vi "UHR-Fleezers Control (host) - Avogadro v2.vi"() -> ()   [LabVIEW 2014] (continued)
  in  "Clear Volume P3":bool caption="Clear Infused Volume"
  in  "Clear Volume P1":bool caption="Clear Infused Volume"
  in  "Display On P1":bool caption="Display On"
  in  "All Pump Parameters":T14={"Pump 1"={"Diameter (mm)"=4.61, "Units"=4.0, "Volume"=100.0, "Rate"=25.0}, "Pump 2"={"Diameter (mm)"=4.61, "Units"=3.0, "Volume"=0.0, "Rate"=0.0}, "Pump 3"={"Diameter (mm)"=4.61, "Units"=4.0, "Volume"=100.0, "Rate"=800.0}}
  in  "Total Volume\nFlushed (uL)":dbl
  in  "Inject Pump 2":bool caption="Inject Pump 2\n(Flush Center)"
  in  "Flush Center Ch Rate (ul/m)":dbl=100.0
  in  "Flush Center Ch Volume (uL)":dbl=15.0
  in  "Pump pause delay (ms)":u32
  in  "Pump write delay (ms)":dbl=300.0
  in  "Ch 3 Inject Rate (ul/h)":dbl=800.0
  in  "Ch 3 Inject Volume (uL)":dbl=100.0
  in  "Ch 1 Inject Volume (uL)":dbl=100.0
  in  "Ch 1 Inject Rate (ul/h)":dbl=25.0
  out "Pump 1 cont disp":string="Right: DNA beads "
  out "Pump 3 cont disp":string="Left: ADig beads"
  in  "Read Harvard":bool
  out "read buffer":string
  out "Serial Settings:Number of Bytes at Serial Port":u32
  in  "write buffer":string
  in  "Tab Control 2":T15(tab)=enum."Feedback on Trap Intensity"
  in  "RF BD 2 to green AOM":bool=TRUE
  in  "RF synth green feedback max":i16=1300
  in  "Phase Increment Trap 2":fxp<+,14,14>=165.0
  in  "Phase offset method":u8=3
  in  "Phase Increment Trap 1":fxp<+,14,14>=165.0
  in  "RF phase reset before cycles":bool
  in  "Update all trap values":bool
  out "Total Counts (ticks)":u16=400
  in  "Trap ON/OFF X or Y Amp?":bool=TRUE
  in  "Oscillate Set 1":bool
  in  "Trap 1 ON":bool=TRUE
  in  "Number Interlace Sets":u8=2 min=1 max=3
  in  "DIO count 3 (ticks)":u16=200
  in  "DIO count 2 (ticks)":u16=200
  in  "DIO count 1 (ticks)":u16=200
  in  "BD 2 Amplitude 3 (%)":dbl min=0.0 max=45.0 step=1.0
  in  "BD 2 Amplitude 2 (%)":dbl min=0.0 max=45.0 step=1.0
  in  "BD 2 Amplitude 1 (%)":dbl min=0.0 max=45.0 step=1.0
  in  "BD 1 Amplitude 3 (%)":dbl min=0.0 max=50.0 step=1.0
  in  "BD 1 Amplitude 2 (%)":dbl=44.0 min=0.0 max=50.0 step=1.0
  in  "BD 1 Amplitude 1 (%)":dbl=45.0 min=0.0 max=50.0 step=1.0
  in  "BD 2 Frequency 3 (MHz)":dbl=26.0 min=0.0 max=40.0 step=0.1 format="%#_6p"
  in  "BD 1 Frequency 3 (MHz)":dbl=70.0 min=60.0 max=90.0 step=1.0 format="%#_6p"
  in  "BD 2 Frequency 2 (MHz)":dbl=26.0 min=0.0 max=40.0 step=0.1 format="%#_6p"
  in  "BD 2 Frequency 1 (MHz)":dbl=26.0 min=0.0 max=40.0 step=0.1 format="%#_6p"
  in  "Not-Interlacing Set":enum32{"Set 1", "Set 2", "Set 3"}(radio)
  in  "Interlace":bool=TRUE
  in  "Trap 2 ON":bool=TRUE
  in  "Trap 3 ON":bool
  in  "Scan axis 2":bool=TRUE
  in  "Osc. amp. (MHz)":dbl=2.0
  in  "Next trap write delay (ticks)":u8
  in  "Manipulation Scaling":cluster{"Horizontal":dbl, "Vertical":dbl}={"Horizontal"=0.075, "Vertical"=0.01}
  out "Coords":T16
  in  "RF amplitude switch delay":u16=2
  in  "BD 1 Delay (ticks)":u8=9
  in  "BD 2 Delay (Ticks)":u8
  in  "Swap F1 and F2":bool
  in  "MCL Step Increment (V_int)":dbl=3.0
  out "Time to Finish All (min)":dbl=0.20000000000000004 format="%#_2p"
  in  "Scan Speed (nm/s)":dbl=50.0
  in  "Scan Range (nm)":dbl=300.0
  in  "Step Size (nm)":dbl=1.0
  in  "MCL/AOM Scale Tweak":dbl=1.0
  in  "MCL Step Position Ratio":dbl=0.5
  in  "Move MCL Also?":bool
  out "Final sep (nm)":dbl=1641.7733990147785
  out "Initial sep (nm)":dbl=1460.0
  out "Save index":dbl=17.0
  out "Final delta (MHz)":dbl=21.477832512315274
  out "Initial delta (MHz)":dbl=20.0
  out "Final freq. (MHz)":dbl=68.52216748768473
  out "Initial freq. (MHz)":dbl=70.0
  in  "Saved AOD Raster Scan Parameter Sets":T17(array[cluster])=[{"Scan Range AOD (nm) 2"=2000.0, "Step Size AOD (nm) 2"=1.0, "Scan Speed AOD (nm/s) 2"=500.0, "Number of scans (AOD) 2"=1, "Label"="offset curve"}, {"Scan Range AOD (nm) 2"=450.0, "Step Size AOD (nm) 2"=1.0, "Scan Speed AOD (nm/s) 2"=100.0, "Number of scans (AOD) 2"=1, "Label"="hp raster check"}, {"Scan Range AOD (nm) 2"=6.8, "Step Size AOD (nm) 2"=0.34, "Scan Speed AOD (nm/s) 2"=0.34, "Number of scans (AOD) 2"=1, "Label"="3.4 kbp - 1 bp steps"}, {"Scan Range AOD (nm) 2"=200.0, "Step Size AOD (nm) 2"=1.0, "Scan Speed AOD (nm/s) 2"=50.0, "Number of scans (AOD) 2"=1, "Label"="dt14 1 14 MHz start"}, {"Scan Range AOD (nm) 2"=450.0, "Step Size AOD (nm) 2"=1.0, "Scan Speed AOD (nm/s) 2"=100.0, "Number of scans (AOD) 2"=1, "Label"="dt14 2 small beads"}, {"Scan Range AOD (nm) 2"=300.0, "Step Size AOD (nm) 2"=1.0, "Scan Speed AOD (nm/s) 2"=100.0, "Number of scans (AOD) 2"=1, "Label"="Oligo"}]
  in  "Load parameters":bool
  out "Scan Range (MHz)":dbl=-1.477832512315271
  in  "Restart DMA? (AOD)":bool=TRUE caption="Restart DMA?"
  out "Incr. int (AOD)":i64=-4701660970
  out "Time/Scan (s) (AOD)":dbl=6.000000000000001 format="%#_2p"
  out "Data points/scans":dbl=1200000.0
  out "Data points/scan (f/b)":dbl=1200000.0
  in  "Save scans":bool=TRUE
  out "AOD Scan I":u64=1 caption="Scan I"
  in  "Continuous AOD Scanning":bool caption="Continuous Scanning"
  in  "Abort AOD Scan":bool caption="Abort Scan"
  in  "Scan BD":bool=TRUE
  out "Cycles/step (AOD)":u64=2000 format="%.3p"
  in  "Number of F/B Scans (AOD)":u16=1 min=1
  out "Scan steps (AOD)":u64=300
  out "Scan Increment (MHz)":dbl=-0.004942583653228331
  out "AOD Scanning":bool caption="Scanning"
  in  "Start AOD Scan":bool caption="Start Scan"
  out "N sets should be saved":dbl=60.0
  out "Progress 2":u16(slide) caption="Progress" scale=0.0..100.0
  in  "Abort save 2":bool caption="Abort save"
  out "MCL Count":dbl=60182.50068666645
  out "T2 feedback amplitude":dbl
  out "T1 feedback amplitude":dbl
  in  "Trap intensity output range":cluster{"Normal High":i16, "Normal Low":i16}={"Normal High"=3000, "Normal Low"=0}
  in  "All FB On/Off":bool
  in  "AI2 to Setpoint":cluster{"Set 1":bool, "Set 2":bool}
  out "AI2 (V)":cluster{"Set 1":dbl, "Set 2":dbl}={"Set 1"=1.9983520004882962, "Set 2"=1.9980468153935362}
  in  "Reset Feedback":cluster{"Set 1":bool, "Set 2":bool}
  in  "Trap Intensity PID Gains":T18={"proportional gain (Kc)"=10, "integral gain (Kc*Ts/Ti)"=5, "derivative gain (Kc*Td/Ts)"=0}
  in  "Feedback On/Off":cluster{"Set 1":bool, "Set 2":bool}={"Set 1"=TRUE, "Set 2"=TRUE}
  out "Actual Setpoint":fxp<+/-,16,1> format="%.16g"
  in  "Dynamic Force FB (ronen)":bool=TRUE
  in  "Remove Unwinding Offset":bool
  in  "Set Reading to\nSetpoint":bool
  out "Trap X (AI1)":T19={"Trap 1"=-0.00103759765625, "Trap 2"=0.0006103515625}
  in  "Trap Pos FB SP":fxp<+/-,16,1>=0.009033203125 caption="Setpoint"
  in  "Trap Pos. FB ON":bool
  in  "Reset Trap Pos. FB":bool
  in  "Tab Control 8":T20(tab)=enum."Dynamic FB settings"
  in  "Red Laser ON/OFF":bool
  in  "Green Laser ON/OFF":bool
  in  "Offset SP2 from SP1":bool
  in  "Use SP 2":bool
  in  "Trap Pos FB Int Count":u16=100
  in  "Trap Pos. FB Gains":T21={"proportional gain (Kc)"=20.0, "integral gain (Kc*Ts/Ti)"=3.0, "derivative gain (Kc*Td/Ts)"=0.0} {"proportional gain (Kc)" format="%.11g"; "integral gain (Kc*Ts/Ti)" format="%.11g"; "derivative gain (Kc*Td/Ts)" format="%.11g"}
  in  "Trap Pos FB SP 2":fxp<+/-,16,1>=-0.10723876953125 caption="Setpoint 2"
  in  "SP2 Offset":fxp<+/-,16,1>=0.100006103515625
  in  "Blue Laser ON/OFF":bool
  in  "Negate Diff?":bool=TRUE
  in  "Differential FB?":bool=TRUE
  in  "Trap Pos. FB Offset Factor":i64
  in  "Trap Pos FB Negate Action":bool=TRUE
  in  "Trap Pos. FB Mult Factor":i64=8388608
  in  "Trap Pos. AI1 X Pre-scale":u16
  in  "Trap Pos. FB Range":T22={"output high"=0.999969482421875, "output low"=-1.0}
  out "Trap Pos FB Int Signal":fxp<+/-,24,9>=0.107635498046875 format="%.18g"
  out "Trap Pos FB Int-Norm Signal":fxp<+/-,16,1>=0.001068115234375 format="%.16g"
  in  "Set SP Using...":bool
  in  "Trap Pos FB Monitor\nT1 or T2":bool
  out "Trap X AI1 (DMA)":T23={"Set 1"=0.001190185546875, "Set 2"=-0.000396728515625}
  in  "N El. to Ave.":dbl=10000.0
  out "Trap Pos FB Action":i64
  in  "Target Force (pN)":dbl
  in  "Read Setpoint Correction File":bool
  out "Offset corrected setpoint":fxp<+/-,17,2>
  in  "Real time Offset file correction for setpoint":bool
  out "B factor":dbl=1.024047487221734
  out "Setpoint offset\ncorrection values":dbl[](array[numeric])=[-0.031124917445190622, -0.030752651903868396, -0.030380386362546155, -0.030008120821223914, -0.0296358552799017, -0.029263589738579454, -0.028891324197257227, -0.02851905865593498, -0.028146793114612746, -0.027774527573290526, -0.027402262031968293, -0.027029996490646066, -0.026657730949323832, -0.02628546540800157, -0.025913199866679372, -0.025540934325357124, -0.025168668784034884, -0.024796403242712664, -0.024424137701390417, -0.024051872160068197, -0.02367960661874595, -0.023307341077423736, -0.02293507553610149, -0.022562809994779262, -0.02219054445345702, -0.021818278912134774, -0.02144601337081256, -0.021073747829490307, -0.02070148228816808, -0.020329216746845853, -0.019956951205523613, -0.019584685664201365, -0.01921242012287913, -0.018840154581556898, -0.01846788904023467, -0.01809562349891245, -0.01772335795759021, -0.017351092416267977, -0.01697882687494575, -0.016606561333623496, -0.01623429579230129, -0.01586203025097902, -0.015489764709656809, -0.015117499168334568, -0.014745233627012341, -0.014372968085690115, -0.014000702544367881, -0.013628437003045626, -0.013256171461723414, -0.01288390592040118, -0.012511640379078946, -0.012139374837756706, -0.011767109296434465, -0.011394843755112245, -0.011022578213790005, -0.010650312672467757, -0.01027804713114553, -0.00990578158982329, -0.009533516048501084, -0.00916125050717883, -0.008788984965856589, -0.008416719424534362, -0.008044453883212128, -0.007672188341889895, -0.007299922800567682, -0.006927657259245414, -0.006555391717923194, -0.00618312617660096, -0.005810860635278733, -0.005438595093956493, -0.005066329552634266, -0.0046940640113120324, -0.004321798469989792, -0.003949532928667565, -0.0035772673873453453, -0.003205001846023084, -0.002832736304700871, -0.0024604707633786305, -0.002088205222056369, -0.0017159396807341423, -0.0013436741394119156, -0.0009714085980896889, -0.000599143056767483, -0.0002268775154452285, 0.00014538802587699823, 0.0005176535671992458, 0.0008899191085214656, 0.00126218464984372, 0.0016344501911659468, 0.0020067157324881735, 0.002378981273810421, 0.0027512468151326547, 0.0031235123564548675, 0.003495777897777108, 0.003868043439099342, 0.004240308980421582, 0.004612574521743823, 0.004984840063066064, 0.005357105604388276, 0.005729371145710531, 0.006101462175864429, 0.006471828951454574, 0.006838267556031237, 0.0071983956637221985, 0.0075492698031555255, 0.007886211739205985, 0.008203425393040836, 0.008495254824253277, 0.008757915090866479, 0.008988509963217262, 0.009185679151985662, 0.009349142811666815, 0.009478823605683882, 0.009575242653604883, 0.009640707437374656, 0.009679768359200001, 0.009697684263568943, 0.009699510091201263, 0.009689446484956905, 0.009670851280319005, 0.009645341636801481, 0.00961482823563782, 0.009581946984451271, 0.009548758869398155, 0.009516624306695143, 0.009486647610544373, 0.00945899676128683, 0.009433027500697355, 0.009406788767248868, 0.009379015134182475, 0.009349965213243244, 0.009319454709649927, 0.009287320976214222, 0.009254311197146217, 0.009220642993305807, 0.009185961068580883, 0.009151064536485683, 0.009117262090596316, 0.009085735431091431, 0.00905816040953128, 0.009036125925089449, 0.009020357076014021, 0.00901100555936031, 0.009008666773597872, 0.009014468451647849, 0.00902903533705348, 0.009052982761144308, 0.009086549802814932, 0.009129160927921771, 0.009179113566578717, 0.00923496835425127, 0.009294711920694344, 0.009355125483714512, 0.009412320729850966, 0.009463946326362715, 0.009510639457078238, 0.009554810019255879, 0.009600031593168357, 0.009650024457447115, 0.00970944742421774, 0.009783743905367674, 0.009878220898935607, 0.00999787326094332, 0.010145165376771278, 0.010317960317968944, 0.010510900903156872, 0.01071768904123823, 0.010932215629711764, 0.011149595024249039, 0.011366640375170052, 0.01158151488223541, 0.011791634767648954, 0.011994506706114787, 0.012190329630524535, 0.012381779837217305, 0.01257149290049768, 0.012760984038198468, 0.012950673146458272, 0.013139710525206412, 0.013327239801665475, 0.013512981370916922, 0.013697234062005528, 0.013879732073992804, 0.01406034909139732, 0.014239542816129637, 0.014417155681788585, 0.014591902654142543, 0.01476237423603835, 0.01492785775256806, 0.015089229385256177, 0.015247537563456863, 0.015404379200532475, 0.015561120295168887, 0.01571638931777187, 0.01586876217297207, 0.016018572183680864, 0.01616652453612384, 0.016313318850516907, 0.016459916919492917, 0.016606514470597182, 0.01675311202170142, 0.016899709572805656, 0.01704630712390992, 0.017192904675014165, 0.017339502226118415, 0.017486099777222666, 0.01763269732832693, 0.01777929487943116, 0.017925892430535433, 0.018072489981639676, 0.018219087532743927, 0.01836568508384817, 0.018512282634952443, 0.018658880186056694, 0.01880547773716093, 0.018952075288265174, 0.019098672839369432, 0.019245270390473683, 0.01939186794157794, 0.0195384654926822, 0.019685063043786435, 0.019831660594890693, 0.01997825814599493, 0.020124855697099202, 0.02027145324820344, 0.020418050799307697, 0.020564648350411954, 0.020711245901516184, 0.020857843452620442, 0.021004441003724693, 0.02115103855482893, 0.0212976361059332, 0.021444233657037445, 0.021590831208141703, 0.02173742875924594, 0.02188402631035022, 0.022030623861454456, 0.022177221412558693, 0.022323818963662957, 0.022470416514767208, 0.022617014065871473, 0.02276361161697571, 0.02291020916807996, 0.023056806719184204, 0.023203404270288462, 0.023350001821392713, 0.023496599372496957, 0.023643196923601208, 0.023789794474705465, 0.023936392025809723, 0.02408298957691396, 0.024229587128018218, 0.02437618467912247, 0.024522782230226726, 0.024669379781330956, 0.024815977332435235, 0.024962574883539465, 0.02510917243464371, 0.025255769985747974, 0.02540236753685222, 0.025548965087956475, 0.025695562639060723, 0.025842160190164994, 0.025988757741269228, 0.02613535529237347, 0.02628195284347773, 0.026428550394581977, 0.026575147945686245, 0.026721745496790485, 0.026868343047894726, 0.027014940598998984, 0.027161538150103234, 0.027308135701207492, 0.02745473325231173, 0.02760133080341599, 0.027747928354520238, 0.027894525905624492, 0.028041123456728743, 0.028187721007832983, 0.028334318558937234, 0.028480916110041495, 0.02862751366114574, 0.028774111212250004, 0.02892070876335424, 0.029067306314458488, 0.02921390386556274, 0.029360501416666993, 0.02950709896777126, 0.029653696518875484, 0.029800294069979756, 0.029946891621084014, 0.030093489172188254, 0.030240086723292495, 0.030386684274396742, 0.030533281825501017, 0.03067987937660525, 0.030826476927709498, 0.03097307447881377, 0.031119672029918, 0.03126626958102226]
  in  "Auto read offset correction":bool=TRUE
  in  "Setpoint Correction Offset File":path=path "C:/Users/Darwin/Desktop/New LabView codes/Thorlabs Motor Codes/Coordinates.txt"
  in  "Semi Passive Mode":bool
  in  "Jump Force (pN)":dbl
  out "Action (%)":dbl(knob) scale=-100.0..100.0
  in  "Trap Pos. FB Out Scale 2^n":u8=23 caption="Action Scale Factor"
  in  "Remove Action Offset":bool
  in  "factor":dbl
  in  "Tab Control 3":enum32{"Timing", "MCL Scan", "Analog Out"}(tab)=enum."MCL Scan"
  in  "Initial Phase Adjustment (APD 3 Gate)":i16=80
  in  "Phase Adj. (APD 3 Gate)":i16=20
  in  "+ phase (APD 3 Gate)":bool
  in  "- phase (APD 3 Gate)":bool
  out "APD 2 Gate Late Counter":u8
  out "APD 2 Gate Relative Phase":i16
  in  "Phase Adj. (APD 2 Gate)":i16=1
  in  "Initial Phase Adjustment (APD 2 Gate)":i16=46
  out "APD 1 Gate Late Counter":u8
  in  "- phase (APD 1 Gate)":bool
  in  "+ phase (APD 1 Gate)":bool
  out "APD 1 Gate Relative Phase":i16
  in  "Phase Adj. (APD 1 Gate)":i16=1
  in  "Initial Phase Adjustment (APD 1 Gate)":i16=46
  in  "Save APD Data\nwith Trap Data":bool=TRUE
  out "APD FIFO Elements Remaining":u32=60
  in  "- phase (APD Acq)":bool
  in  "+ phase (APD Acq)":bool
  out "APD Acq Late Counter":u8
  out "APD Acq Relative Phase":i16
  in  "Phase Adj. (APD Acq)":i16=20
  in  "Initial Phase Adjustment (APD Acq)":i16
  in  "Invert APD Gate":bool caption="Invert Gate"
  in  "APD Gate OFF Count":u16=450 caption="Gate OFF Count"
  in  "APD Gate ON Count":u16=150 caption="Gate ON Count"
  in  "APD Gate":enum32{"ON", "OFF", "Interlace"}(radio)=enum."Interlace"
  in  "APD Integration Time (s)":dbl=0.001 caption="Integration Time (s)"
  out "APD Acq Rate (Hz)":dbl=1000.0 caption="Rate (Hz)"
  out "APD Samples/FIFO Acq.":dbl=200.0 caption="Single APD Samples/DMA read"
  out "APD Elements/DMA read":u32=600 caption="All APD Elements/DMA read"
  out "APD Int. Count":u32=40000 format="%.0p"
  in  "+ phase (APD 2 Gate)":bool
  in  "- phase (APD 2 Gate)":bool
  out "APD 3 Gate Late Counter":u8
  out "APD 3 Gate Relative Phase":i16
  out "Number of APDs":u8=3
  in  "Tab Control 5":enum32{"PSD X", "PSD Y", "Other Data Channel"}(tab)=enum."Other Data Channel"
  out "Data map":dbl[][](graph)=[[-0.048833919859841396, -0.04562305134849659, -0.034945824689939016, -0.03856523007204608, -0.04332584499952716, -0.03705651703387691, -0.03441193823145684, -0.03447728939721072, -0.03398020997038663, -0.03203982097634292, -0.028964547258383322, -0.027133282250795705, -0.02402369458347961, -0.022370810606792614, -0.02285208541427248, -0.022022892519572453, -0.017491715558080566, -0.028058484144828894, -0.024438753971776583, -0.020884668157221772], [-0.044858343864006875, -0.04750505026346981, -0.04373283633504831, -0.04118626507163741, -0.04512151651670596, -0.03609855082525881, -0.033744697137220614, -0.03367065821277415, -0.03224206961429411, -0.0280300824268187, -0.03176369177394743, -0.027681526439645908, -0.030236105063729535, -0.025280934517311407, -0.022191013313833257, -0.027728213969859677, -0.018010469311187872, -0.02053182051646974, -0.018905379569266585, -0.017046838486900306], [-0.04619265839121586, -0.038666821391394615, -0.04063200878963933, -0.038870918291910306, -0.038253708890616, -0.04121933117813677, -0.036986543894992875, -0.028687142808565654, -0.0324931227248371, -0.02779123369663754, -0.029391511058635078, -0.027480848639991888, -0.02796901729268089, -0.028052879851808054, -0.023474727560020767, -0.023950199933010848, -0.017939033842884144, -0.02402621581006516, -0.019419161851830506, -0.026130138109084128], [-0.044893648826491675, -0.038593543996048155, -0.034920168730450216, -0.04273432165883133, -0.04450442864203366, -0.03912189883341463, -0.03756864818035341, -0.03081041675402709, -0.03297657507462223, -0.02983645523075837, -0.030290202478222082, -0.027336078388796602, -0.0254889070719212, -0.02822716191191465, -0.022648458602810895, -0.029554000947954604, -0.023868769278601577, -0.02707397500210064, -0.021218877084591012, -0.023390621058401683], [-0.03792125563439862, -0.035917871520177384, -0.03584124706409223, -0.03467748614293901, -0.037177622486417775, -0.04054489615935812, -0.032135985275886646, -0.0359415435337013, -0.03316432300305255, -0.03345865514511251, -0.028443324349092167, -0.027305480285792286, -0.026528386416700064, -0.027264811807360866, -0.029569080226431475, -0.02743184215872684, -0.0251592402424164, -0.02578413565975518, -0.01933358430626013, -0.021580686396973428], [-0.03741733191068357, -0.03802342249748768, -0.03301932709885415, -0.032878699946914634, -0.03636258670854889, -0.03801428975937023, -0.035499778738436044, -0.03366566459479707, -0.03267063244235234, -0.031994556278940794, -0.031958207900763064, -0.029583753635326074, -0.029472698610106388, -0.028001618188858123, -0.027660463315929855, -0.02837908598592112, -0.02876035056394463, -0.028306656123681804, -0.022532147026323075, -0.020076155502178426], [-0.03852704945038462, -0.03706418529940301, -0.034830754540261605, -0.03081036506808769, -0.029973739636454205, -0.03465115042102995, -0.03519548731668977, -0.03254535288059757, -0.032203324283535804, -0.03117997679069996, -0.02796070219331038, -0.02869747864544056, -0.03316171349305196, -0.029868059194884514, -0.02612470174756419, -0.027292619822721347, -0.031143517406971726, -0.013026310002840815, -0.018050660566856974, -0.02200311497108313], [-0.026939570662517315, -0.03633812603684408, -0.028073392405746217, -0.03189486982397553, -0.025130436130217745, -0.03375323568423947, -0.031322462311797895, -0.03210024464047708, -0.02810983769169843, -0.030051376454254312, -0.029112296808817967, -0.025447236839430763, -0.030207552424648558, -0.030867162390747615, -0.024498891313261502, -0.027036942531945482, -0.027463597754890705, -0.0222543010934024, -0.025184873838279498, -0.02245763543126285], [-0.031694705376812196, -0.03268856164273058, -0.02952947063909147, -0.029735520736915468, -0.02544825753451345, -0.030562742944417846, -0.02701472752214199, -0.029917776201167187, -0.02616036846939392, -0.02771389778838171, -0.02186210577962481, -0.024121417503406007, -0.030437442210848036, -0.02448871788986926, -0.02590267265143363, -0.024035501151775992, -0.024162793276532854, -0.015138321922208507, -0.020610761507581794, -0.019783363192404497], [-0.025170433111853244, -0.02644722457505009, -0.03065248600223553, -0.03340126076134131, -0.028587965486493117, -0.03408763168204955, -0.02990101362824416, -0.025992643031853717, -0.028244300308286778, -0.028070839023166108, -0.0219881312643384, -0.02368338305394878, -0.029203010967967805, -0.0246296388600473, -0.022648036472129887, -0.02271203678985071, -0.025879899474311702, -0.012361408705672077, -0.02113464565426776, -0.01637086989336777], [-0.019556684854486167, -0.028508825307830006, -0.027410697844203386, -0.02572867351545044, -0.023132008681563912, -0.029827675734389207, -0.020226381795655134, -0.02750616071425497, -0.02019952240975257, -0.020934320671278525, -0.02340424884694765, -0.02059822765424934, -0.025858902232121297, -0.021866132000065906, -0.02045015744837099, -0.020480394072565463, -0.02096860624850998, -0.01350265027550329, -0.018607583704501007, -0.011697664042299171], [-0.02182526688820388, -0.029272696479715057, -0.02191052144669742, -0.025109075938590235, -0.02251871946068537, -0.029046450694127472, -0.024447507647804553, -0.02327792964162035, -0.023803104497111593, -0.023473739519855905, -0.017180547955894195, -0.016320152050817407, -0.0215906299531042, -0.022871472134949992, -0.0198512961194604, -0.008532123268847187, -0.018260170448214954, -0.011304000794752432, -0.015532769706513346, -0.007211589509415313], [-0.02058204704527899, -0.02682225934681356, -0.016875902015732528, -0.016252765288678583, -0.017702085327042694, -0.024635448511257357, -0.01824678580937727, -0.01979393689765926, -0.01902201210524649, -0.01936247429699857, -0.01739236956106093, -0.01758753812992196, -0.018160054261808112, -0.015598043317867523, -0.018297114524111712, -0.009884245824658567, -0.011791400689120471, -0.011487479907455737, -0.01072072071265525, -0.007451956455915898], [-0.02280961986658019, -0.01871923144869239, -0.019504783623135263, -0.021972581104426663, -0.01901917955358607, -0.019027286069886205, -0.018270257028251996, -0.018596587273849018, -0.016709037632870405, -0.017697057473102438, -0.014978575669980457, -0.010603203337063225, -0.013642564827630287, -0.012917892682123904, -0.013298786535371122, -0.0049432166322443, -0.011174949650270499, -0.004720443717086445, -0.011459013596701543, -0.0016791139598016924], [-0.018650910305237373, -0.016357147152896795, -0.018162350922211336, -0.024238632218878096, -0.011862016875947182, -0.01684013245324201, -0.018218312089914424, -0.015766086559833793, -0.008923780168161085, -0.017342433376067078, -0.00982670552699491, -0.007485834838981667, -0.011581612699895726, -0.010499689109418502, -0.008061683169760516, -0.0009263556671392408, -0.008565317713788972, -0.0027868438284506664, -0.009844722696513451, -0.0019210712903448826], [-0.02267870167657219, -0.01820567945642372, -0.015553541835574405, -0.01816081385036544, -0.013758641541072114, -0.0150976770403269, -0.007420756672035633, -0.013389246549250933, -0.006514958926164554, -0.006462841128412328, -0.00952435808067929, -0.00475069398470615, -0.00459707774563671, -0.005308995802270828, -0.008730344274091627, 0.002731514013538985, -0.002868980157839535, -0.0022046930339780953, -0.005056814086691998, -0.0007670178572610417], [-0.017689364706836717, -0.015925902357021578, -0.015144016111471186, -0.016540584512005983, -0.013351277392059047, -0.013943443477761453, -0.010191656677240805, -0.014447687845507007, -0.008294883809384005, -0.004006535139136523, -0.004602354254100462, -0.005708147329809433, 0.0010905745261097916, -0.0013363437553225981, -0.005142447810681263, 0.0014330503733632552, -0.00035962634572572934, 0.0006370803646549156, -0.002343381389865588, 0.00646713880908097], [-0.016900021051424876, -0.016443355701240392, -0.015377983185878207, -0.010020245136092634, -0.0066416379496751, -0.011613172317058176, -0.0053077128094028364, -0.006205329222632868, -0.001430736757324482, -0.00293391346514837, 0.00010158552007738346, -0.0018697192264156108, 0.003508214972856638, 0.002553390392833331, -0.004562064348932344, -0.001624381209515205, 0.004340196861586832, 0.0009744857396142472, 0.006375862997116909, 0.005585046094750511], [-0.01596336781117824, -0.011702818300753287, -0.010916504253215015, -0.009254345679262128, -0.008604075095927748, -0.0018924670019224953, -0.00855333040348221, -0.010447290327726972, 0.003261724825270835, 0.0009009772684124171, 0.004051926290892741, 0.0021880308767305767, 0.006041746656433683, 0.008425761635750241, 0.0014453528605402402, 0.004178755736227903, 0.005780081838197235, 0.006264646335816101, 0.0037995923748903645, 0.005044674210819564], [-0.011164162935648118, -0.011909093650055576, -0.007164005040066388, -0.0033160708755370265, -0.0019808929991613116, -4.6568041219333806e-05, -0.005030950798490225, -0.002035897955447696, 0.0009148203582524921, 0.0034381005552099825, 0.005071258907286298, 0.003987492148758313, 0.002458665648117312, 0.007332034034771947, 0.0013924095874078349, 0.0011400204241978802, 0.01235003101109109, 0.006919585826940114, 0.006725745076626429, 0.0013723081089635023], [-0.0062451800040877175, -0.00022724780683755583, -0.007287178588684788, 0.0004107315285382096, -0.0015013075078963165, -0.0012779837579695672, -0.002757151360555635, 0.00038145257000220256, 0.0010617715834819342, 0.011860583343293013, 0.004211760981532914, 0.007675718015663701, 0.006950284168949206, 0.002455711840427803, 0.005437443029862904, 0.0010348857063814665, 0.009694647230553532, 0.009881701746196906, 0.008987174271975774, 0.007448751229657158], [-0.002579647264833691, 0.003437689956020563, 0.0011802771839093179, -0.0013727640378685922, 0.007495384319305234, 0.004596393912357324, 0.0019146546803592412, 0.004935323360582491, 0.004287176488907663, 0.00955592382246558, 0.008765648956954898, 0.006319787866766563, 0.0022380698379930366, 0.0075011672254434135, 0.004387389677744142, 0.007438410924317888, 0.010749603863094722, 0.00667338644975694, 0.013000957496797076, 0.005390884988364584], [-0.0016043140430406421, 0.00103032454634755, -0.0022551769660642254, 0.004300495959151877, 0.007004511828609751, 0.008090128765368618, 0.00027502130979898797, 0.009750828259516542, 0.004547686672545811, 0.005567346910242144, 0.011033323451339328, 0.009736807436815771, 0.004430018541283793, 0.007718633367189761, 0.005533825044168685, 0.008161459568885122, 0.010361358736629323, 0.00643089454478096, 0.014868015137623076, 0.0066910722261343866], [0.0021890976433014764, 0.007846604465446834, 0.00447742426107851, 0.006768968130770921, 0.009115402720418017, 0.006826167285019172, 0.008294010687113156, 0.01322999272888498, 0.011132998783167475, 0.0029311543331256773, 0.013063553990137632, 0.01305907774440814, 0.005019961404667499, 0.007368331669566155, 0.016594840092172887, 0.012930947160349818, 0.006272513382154017, 0.006702691443599395, 0.016184872256304612, 0.008851297838506371], [0.005011638961224373, 0.0076441728747117695, 0.00621355125980238, 0.01061231408622043, 0.012381414949437428, 0.011203338514464103, 0.010884424071649627, 0.017218793424435046, 0.015983341227086497, 0.011067063607259075, 0.014777786899572333, 0.012060539657579972, 0.0100983446166572, 0.006256936865974087, 0.01323545088680157, 0.010094576800794968, 0.008615433745884402, 0.008479368717686595, 0.012238018722461164, 0.009772149298620254], [0.006145128667572415, 0.009583124190721524, 0.008230210814216425, 0.012770015962521487, 0.0072401700214171335, 0.01792433719205669, 0.013001552239716706, 0.019793863973321037, 0.016731176702518714, 0.0124363611091214, 0.02085801251584035, 0.01790623805109556, 0.011413884933645407, 0.009214773559537454, 0.019123999628382085, 0.013596253708872113, 0.011085725395278826, 0.013006606648484869, 0.014473123497119832, 0.01187288948713287], [0.008450591124271604, 0.012452734948455769, 0.010730177687075518, 0.015034201932504956, 0.016300084936743866, 0.017550925667482002, 0.01540434027769054, 0.018058057775796138, 0.018605285156422072, 0.018682555998842103, 0.019089915919035992, 0.02023124093592352, 0.017680813546864987, 0.014937003501406414, 0.024937406998947774, 0.01414608431184411, 0.014331875159052022, 0.015010134466561744, 0.019319364154556116, 0.008956207509970494], [0.015758080955936164, 0.008146837382692257, 0.01482027810490209, 0.018573503666719598, 0.02070995054212195, 0.017633689578998177, 0.01868235815075362, 0.01604488675196563, 0.014836673918363272, 0.026669639135622196, 0.021377178985350548, 0.023647500993477732, 0.019698096234492743, 0.018791720238891117, 0.023283487172617766, 0.019587853878651935, 0.019972116701210484, 0.012020640293795138, 0.018764177181255084, 0.010789103723526334], [0.015269094489419675, 0.010943473849416465, 0.016221346219908804, 0.019666975295993237, 0.020087505364799554, 0.01371466888924022, 0.021745103795755803, 0.024754317609140573, 0.02360238946651743, 0.025207800521040803, 0.025912245852829457, 0.02675226516415067, 0.027445903482807003, 0.024839997524446825, 0.025091702049854718, 0.021287738733215312, 0.018354248722045618, 0.018329615643996124, 0.021389929189533256, 0.02049148018889178], [0.017908555764461244, 0.013686583464181785, 0.01885352797745572, 0.019643969643496483, 0.020226869605798024, 0.02121808112821011, 0.03037704758431377, 0.024574136522770594, 0.025106830457833497, 0.0322324105979884, 0.028461351755605557, 0.02622152588965411, 0.02347280325457083, 0.026209940937467063, 0.02619273745496397, 0.022756883831864035, 0.02089981804840832, 0.024736288994078336, 0.019599605505547443, 0.0198630434690626], [0.013983900555606988, 0.019498333151302602, 0.028058383894891074, 0.022568671668644104, 0.02696903555948043, 0.022715045246434622, 0.029288792803816778, 0.02967619779854612, 0.030569028236382814, 0.03245623448948691, 0.028056370253880004, 0.029463694650405797, 0.023747280613036083, 0.03083625385354659, 0.031651878669780406, 0.028628506027632762, 0.02249608142107653, 0.024620626769190912, 0.02363922792816043, 0.02864126784216391], [0.01822222075736896, 0.022634871598822652, 0.020539712709323844, 0.021911949037495472, 0.02530760172363056, 0.02470854648688484, 0.03644209017029453, 0.026279678616177957, 0.027319968931289892, 0.03273898376621685, 0.034837500674306444, 0.030676362882715184, 0.02746391323684006, 0.031862700415465885, 0.03023056525850469, 0.025411914201329208, 0.02884732666297697, 0.027364916126284094, 0.026849878868070765, 0.03159153646398022], [0.019633223296338494, 0.02542321951626408, 0.02909024874098195, 0.030107489456354095, 0.02566876859575037, 0.028751129008875533, 0.031475722366085715, 0.028794597148901025, 0.028773532962156245, 0.03610482220746554, 0.03153666588075027, 0.030515146443015194, 0.03444020061998032, 0.03346147734988518, 0.028644767651394197, 0.031131371599984612, 0.031986031871811565, 0.03130436775549575, 0.028363302816391274, 0.037600905614623606], [0.022048465940376016, 0.024314126907380853, 0.03394149568939957, 0.025511281297002773, 0.030395141953679573, 0.03172877923065929, 0.033901299212516965, 0.02307378095022041, 0.03218289999487623, 0.03300158160378726, 0.03708023163987077, 0.03658233192167528, 0.034601992286632244, 0.0354911572893855, 0.030442878914396627, 0.04386142219038186, 0.029538237308558885, 0.036048325671956816, 0.027464674946100068, 0.037636826950737085], [0.027051212397025022, 0.029685693195531798, 0.026162622506224073, 0.02663502575091299, 0.0330034373720801, 0.03772159407988603, 0.04103768587131309, 0.028794707082410713, 0.034467735033289454, 0.03171115045183262, 0.035618050634250484, 0.03599108706256059, 0.038413412955178576, 0.036131713813920135, 0.03417132251890828, 0.02910773819389756, 0.033868663984601366, 0.03423377043721337, 0.030199857055129477, 0.038535521422790264], [0.028491631032645112, 0.03222684711514713, 0.02849596685422396, 0.028881266268511053, 0.030719412057483166, 0.029378947232053927, 0.03364314304800326, 0.03190085472591245, 0.032856841742297235, 0.034241530079825964, 0.03618090414256477, 0.03771375682099936, 0.03326717501037413, 0.038271010725054205, 0.03311204802387357, 0.03902193760899049, 0.03598577063425182, 0.03510523686979037, 0.03390952760171352, 0.04025668538983444], [0.0313920662628196, 0.03138494480639911, 0.03080999873345397, 0.027820476816305985, 0.03636247399009268, 0.03664473547682157, 0.030727492794039874, 0.031163688203649044, 0.03423413138290959, 0.032837149859900466, 0.031142202142960235, 0.04236914345556958, 0.0385007046079337, 0.039961259497033455, 0.03548485866141547, 0.038209982759363645, 0.03843389187207174, 0.03473846283224203, 0.02905997046639896, 0.03723266150091976], [0.028601475312463816, 0.0320975444707591, 0.030982050904848346, 0.02983897184607335, 0.035838815584353395, 0.03916844364472581, 0.031695007811736606, 0.031733095315208744, 0.03816165021700833, 0.04041260420766596, 0.033038901620110694, 0.03760382929867345, 0.036887027143281, 0.037295388937902074, 0.03605361320563879, 0.039708209814781924, 0.03476390641213979, 0.03154209943008692, 0.02858339364248484, 0.034195850855496174], [0.0374761670639246, 0.03243086722540377, 0.030563175175887358, 0.028416490962318137, 0.034115152700655044, 0.03231904375567549, 0.034317341913455264, 0.03066989410977178, 0.03837979435410121, 0.03906485199796114, 0.03477180720467114, 0.035059916701733806, 0.040043271749882585, 0.040346932391163395, 0.03374691778190896, 0.03816314782383155, 0.036481943094579646, 0.03698557454848565, 0.02995702546333101, 0.034904637665734664], [0.022513271758968167, 0.03545278208740031, 0.028902878027849684, 0.031113620492952306, 0.03551965495900841, 0.03158178942706804, 0.03691460424262337, 0.03344578060185349, 0.037446582486708575, 0.035860756950936094, 0.03098162756853649, 0.037897545991919954, 0.04264330302423301, 0.04395788246909649, 0.03785544020883423, 0.03723687052847083, 0.037230958732163325, 0.03176469556416903, 0.03408205014677066, 0.029756103596108238]]
  in  "Channel":i32=4
  in  "Abort MCL Scan":bool
  out "MCL Scan I":u64
  out "MCL Scanning":bool
  in  "Start MCL Scan":bool
  out "wait to reset values":bool
  in  "Tab Control 4":enum32{"Scan Settings", "MCL FPGA Loop Timing"}(tab)
  out "Total Time (s)":dbl=4.8
  in  "Scan lines (y)":u64=20
  in  "Fast Scan Dir":bool=TRUE
  in  "2D or 1D Scan":bool=TRUE
  out "Initial X":dbl=-1.499252296517838
  out "Initial Y":dbl=-0.7047639393292031
  out "Time/f+b scan (s) (MCL)":dbl=0.24 caption="Time/scan (s)"
  in  "Number of scans (MCL)":u64=1 caption="Scans"
  in  "Scan steps (MCL)":u64=40 caption="Scan steps (x)"
  in  "N APD Samp/step":dbl=3.0
  in  "Scan Range (V)\n(of steps)":dbl=7.0
  in  "Restart DMA? (MCL)":bool=TRUE caption="Restart DMA?"
  in  "Continuous MCL Scanning":bool caption="Cont. Scanning"
  in  "Center Scan":bool=TRUE
  in  "Save Data (MCL)":bool=TRUE caption="Save Data"
  out "Actual Incr. int (MCL)":i16=588 caption="Incr. int"
  out "Desired incr (int)":dbl=588.125641025641
  out "Desired Scan Incr (V)":dbl=0.1794871794871795
  out "N sets should be saved (MCL)":dbl=24.0 caption="N sets should be saved"
  out "Data points/scans (MCL)":dbl=4800.0 caption="Data points/scans"
  out "Data points/scan (f+b)":dbl=240.0 caption="points/scan (f+b)"
  out "Cycles/step (MCL)":u64=300 caption="Cycles/step" format="%.0p"
  out "Actual MCL Inc (V)":dbl=0.1794488357188635
  in  "Phase adjust (MCL)":i16 caption="Phase adjust"
  out "Relative Phase (MCL)":i16 caption="Relative Phase"
  in  "Initial Phase Adj. (MCL)":i16 caption="Initial Phase Adj."